vi "Dresden R2R Sputter 03.02.2018 IY24.vi"() -> ()   [LabVIEW 2009] (continued)
      tunnel: w5831 -> [w5835 w5844]
      tunnel: [w5835 w5842] -> w5828
      tunnel: w5830 -> [_ w5843]
      frame #0 {
      }
      frame #1 {
        n4043 = local read "Roll Status"() -> (w5841:T1)
        n4044 = Multiply(x=9.3, y=3.141592653589793) -> (x*y=w5838:dbl)
        n4045 = Multiply(x="RPM", y=6) -> (x*y=w5847:dbl)
        n4046 = Divide(x=w5843, y=u32 1000 ("milliseconds to wait")) -> (x/y=w5846:dbl)
        n4047 = Multiply(x=w5838, y="RPM") -> (x*y=→"Cevre":dbl)
        n4048 = Multiply(x=w5847, y=w5846) -> (x*y=w5845:dbl)
        n4049 = case shown="\"Backward\"" w5841 {
          tunnel: w5845 -> [w5856 w5863]
          tunnel: w5844 -> [w5855 w5862]
          tunnel: [w5852 w5857] -> w5842
          frame #0 {
            n4050 = Subtract(x=w5855, y=w5856) -> (x-y=w5851:dbl)
            n4051 = Less?(x=w5851, y=0.0) -> (x < y?=w5854:bool)
            n4052 = Select(t=360.0 ("y"), s=w5854, f=w5851) -> (s? t:f=w5852:dbl)
          }
          frame #1 {
            n4053 = Add(x=w5862, y=w5863) -> (x+y=w5858:dbl)
            n4054 = Less?(x=360.0 ("y"), y=w5858) -> (x < y?=w5861:bool)
            n4055 = Select(t=0.0 ("y"), s=w5861, f=w5858) -> (s? t:f=w5857:dbl)
          }
        }
      }
    }
    "Angle" <- w5828
    "Gauge" <- w5828
    n4056 = local read "Sim"() -> (w5829:bool)
  }
  n4057 = call <vilib>:"Read JPEG File.vi"("path to JPEG file"=w397) -> ("image data"=w396:T34)  [unwired: 8 in, 2 out]
  n4058 = call <vilib>:"Read JPEG File.vi"("path to JPEG file"=w398) -> ("image data"=w399:T34)  [unwired: 8 in, 2 out]
  n4059 = call <vilib>:"Read JPEG File.vi"("path to JPEG file"=w407) -> ("image data"=w406:T34)  [unwired: 8 in, 2 out]
  n4060 = call <vilib>:"Read JPEG File.vi"("path to JPEG file"=w313) -> ("image data"=w314:T34)  [unwired: 8 in, 2 out]
  n4061 = Build Path(base path="Gui_ch2_front_path", name or relative path="bv3 fail.jpg") -> (appended path=w114:path)
  n4062 = while {
    tunnel: w17 -> [w5874]
    tunnel: w16 -> [w5873]
    tunnel: [w5880] -> w15
    tunnel: [w5879] -> w14
    tunnel: data[3B] ("Serial Parameters") -> [w5868]
    stop <- FALSE stop-if-true
    # "Haberlesmenin sadece gerekli olan degerler ile\ndegilde tum degerler ile yapilmis olmasi\nhaberlesme hizini dusuruyor olabilir."
    n4063 = disable-structure shown="Enabled" {
      disable-tunnel: [w5912 w5934] -> w5877
      disable-tunnel: [w5911 w5936] -> w5876
      disable-tunnel: [w5910 w5938] -> w5875
      disable-tunnel: w5874 -> [w5909 w5947]
      disable-tunnel: w5873 -> [w5908 w5945]
      disable-tunnel: [w5907 w5944] -> w5872
      disable-tunnel: [w5906 w5946] -> w5871
      disable-tunnel: [w5905 w5948] -> w5870
      disable-tunnel: "Sim" -> [w5904 _]
      disable-tunnel: w5868 -> [w5903 w5948]
      disable-tunnel: [w5902 w5940] -> w5864
      frame #0 {
        n4064 = case shown="True" w5904 {
          tunnel: [w5928 "Sensor_DI Sim"] -> w5912
          tunnel: [w5927 "Sensor_DI Sim"] -> w5911
          tunnel: [w5926 "Sensor_DI Sim"] -> w5910
          tunnel: [w5925 "Sensor_DI Sim"] -> w5902
          tunnel: w5909 -> [w5924 w5932]
          tunnel: w5908 -> [w5923 w5931]
          tunnel: [w5922 w5931] -> w5907
          tunnel: [w5921 w5932] -> w5906
          tunnel: [w5913 w5929] -> w5905
          tunnel: w5903 -> [w5913 w5929]
          frame #0 {
            n4065 = call-poly <vilib>:"MB Serial Master Query (poly).vi"("VISA resource name"=w5924, "Starting Address"=u16 8, "Quantity"=u16 4, "error in"=w5923, "Serial Parameters"=w5913) -> ("VISA resource name out"=w5921:refnum<visa-resource-name>, "Discrete Inputs"=w5920:bool[], "error out"=w5922:errorcluster)  [unwired: 1 in, 11 out]
            n4066 = Index Array(array=w5920, index=0) -> (element=w5925:bool)
            n4067 = Index Array(array=w5920, index=1) -> (element=w5926:bool)
            n4068 = Index Array(array=w5920, index=2) -> (element=w5927:bool)
            n4069 = Index Array(array=w5920, index=3) -> (element=w5928:bool)
          }
          frame #1 {
          }
        }
      }
      frame #1 {
        n4070 = local read "Ch3_Motor_DO"() -> (→"Ch1_SRV_start_stop_do":bool)
        n4071 = call-poly <vilib>:"MB Serial Master Query (poly).vi"("VISA resource name"=w5947, "Starting Address"=u16 0, "Quantity"=u16 4, "error in"=w5945, "Serial Parameters"=w5948) -> ("VISA resource name out"=w5946:refnum<visa-resource-name>, "Discrete Inputs"=w5933:bool[], "error out"=w5944:errorcluster)  [unwired: 11 in, 1 out]
        n4072 = Index Array(array=w5933, index=3) -> (element=w5934:bool)
        n4073 = Index Array(array=w5933, index=2) -> (element=w5936:bool)
        n4074 = Index Array(array=w5933, index=1) -> (element=w5938:bool)
        n4075 = Index Array(array=w5933, index=0) -> (element=w5940:bool)
      }
    }
    "Ch1_Sensor_DI" <- w5864
    "Ch4_Sensor_DI" <- w5877
    "Ch2_Sensor_DI" <- w5875
    "Ch3_Sensor_DI" <- w5876
    "Ch1_SRV1_counter_di" <- w5864
    n4076 = Wait (ms)(milliseconds to wait=u32 5) -> ()  [unwired: 1 out]
    n4077 = local write "Sensor_DI Sim"(w5864) -> ()
    n4078 = disable-structure shown="Enabled" {
      disable-tunnel: "Ch1_Motor_DO" -> [w5893 w5900]
      disable-tunnel: [w5889 w5896] -> w5880
      disable-tunnel: [w5888 w5895] -> w5879
      disable-tunnel: w5872 -> [w5885 w5897]
      disable-tunnel: w5871 -> [w5884 w5898]
      disable-tunnel: w5870 -> [w5883 w5899]
      frame #0 {
        n4079 = Build Array(w5893, "Ch2_Motor_DO", "Ch3_Motor_DO", "Ch4_Motor_DO", "Motor_Dir_DO") -> (w5891:bool[])
        n4080 = call-poly <vilib>:"MB Serial Master Query (poly).vi"("VISA resource name"=w5884, "Starting Address"=u16 320, "Coils"=w5891, "error in"=w5885, "Serial Parameters"=w5883) -> ("VISA resource name out"=w5889:refnum<visa-resource-name>, "error out"=w5888:errorcluster)  [unwired: 12 in, 1 out]
      }
      frame #1 {
        n4081 = call-poly <vilib>:"MB Serial Master Query (poly).vi"("VISA resource name"=w5898, "Address"=u16 320 ("Starting Address"), "Coil"=w5900, "error in"=w5897, "Serial Parameters"=w5899) -> ("VISA resource name out"=w5896:refnum<visa-resource-name>, "error out"=w5895:errorcluster)  [unwired: 12 in, 1 out]
      }
    }
    n4082 = call "Elapsed Time145"() -> ("Elapsed Time (s)"=w5865:dbl)  [unwired: 12 in, 7 out]
    n4083 = feedback #121() -> (w5866:dbl)  [unwired: 1 in]
    n4084 = Subtract(x=w5865, y=w5866) -> (x-y=→"COM12 Loop Time":dbl)
  }
  n4085 = call <vilib>:"Read JPEG File.vi"("path to JPEG file"=w300) -> ("image data"=w299:T34)  [unwired: 8 in, 2 out]
  n4086 = call <vilib>:"Read JPEG File.vi"("path to JPEG file"=w410) -> ("image data"=w411:T34)  [unwired: 8 in, 2 out]
  n4087 = call <vilib>:"Read JPEG File.vi"("path to JPEG file"=w310) -> ("image data"=w309:T34)  [unwired: 8 in, 2 out]
  n4088 = Build Path(base path="Gui_ch2_front_path", name or relative path="bv3 on.jpg") -> (appended path=w117:path)
  n4089 = call <vilib>:"Read JPEG File.vi"("path to JPEG file"=w303) -> ("image data"=w304:T34)  [unwired: 8 in, 2 out]
  n4090 = Build Path(base path="Gui_ch2_top_path", name or relative path="atm3 fail.jpg") -> (appended path=w249:path)
  n4091 = Build Path(base path="Gui_ch2_front_path", name or relative path="gv front failled2.jpg") -> (appended path=w227:path)
  n4092 = call <vilib>:"Read JPEG File.vi"("path to JPEG file"=w106) -> ("image data"=w107:T34)  [unwired: 8 in, 2 out]
  n4093 = call <vilib>:"Read JPEG File.vi"("path to JPEG file"=w365) -> ("image data"=w364:T34)  [unwired: 8 in, 2 out]
  n4094 = call <vilib>:"Read JPEG File.vi"("path to JPEG file"=w149) -> ("image data"=w150:T34)  [unwired: 8 in, 2 out]
  n4095 = Build Path(base path="Gui_ch2_top_path", name or relative path="atm3 on.jpg") -> (appended path=w250:path)
  n4096 = Build Path(base path="Gui_ch2_top_path", name or relative path="pg2 fail.jpg") -> (appended path=w254:path)
  n4097 = Build Path(base path="Gui_ch2_top_path", name or relative path="cc fail.jpg") -> (appended path=w261:path)
  n4098 = Build Path(base path="Gui_ch2_top_path", name or relative path="pg2 fail.jpg") -> (appended path=w267:path)
  n4099 = call <vilib>:"Read JPEG File.vi"("path to JPEG file"=w473) -> ("image data"=w472:T34)  [unwired: 8 in, 2 out]
  n4100 = call <vilib>:"Read JPEG File.vi"("path to JPEG file"=w477) -> ("image data"=w478:T34)  [unwired: 8 in, 2 out]
  n4101 = Build Path(base path="Gui_ch2_top_path", name or relative path="pg2 on.jpg") -> (appended path=w253:path)
  n4102 = Build Path(base path="Gui_ch2_top_path", name or relative path="cc on.jpg") -> (appended path=w262:path)
  n4103 = Build Path(base path="Gui_ch2_top_path", name or relative path="pg2 on.jpg") -> (appended path=w268:path)
  n4104 = call <vilib>:"Read JPEG File.vi"("path to JPEG file"=w103) -> ("image data"=w102:T34)  [unwired: 8 in, 2 out]
  n4105 = call <vilib>:"Read JPEG File.vi"("path to JPEG file"=w537) -> ("image data"=w536:T34)  [unwired: 8 in, 2 out]
  n4106 = call <vilib>:"Read JPEG File.vi"("path to JPEG file"=w368) -> ("image data"=w369:T34)  [unwired: 8 in, 2 out]
  n4107 = call <vilib>:"Read JPEG File.vi"("path to JPEG file"=w487) -> ("image data"=w488:T34)  [unwired: 8 in, 2 out]
  n4108 = call <vilib>:"Read JPEG File.vi"("path to JPEG file"=w474) -> ("image data"=w475:T34)  [unwired: 8 in, 2 out]
  n4109 = call <vilib>:"Read JPEG File.vi"("path to JPEG file"=w146) -> ("image data"=w145:T34)  [unwired: 8 in, 2 out]
  n4110 = Build Path(base path="Gui_ch2_top_path", name or relative path="bv1 fail.jpg") -> (appended path=w272:path)
  n4111 = Build Path(base path="Gui_ch2_front_path", name or relative path="gv front open2.jpg") -> (appended path=w230:path)
  n4112 = call <vilib>:"Read JPEG File.vi"("path to JPEG file"=w538) -> ("image data"=w539:T34)  [unwired: 8 in, 2 out]
  n4113 = call <vilib>:"Read JPEG File.vi"("path to JPEG file"=w527) -> ("image data"=w526:T34)  [unwired: 8 in, 2 out]
  n4114 = call <vilib>:"Read JPEG File.vi"("path to JPEG file"=w499) -> ("image data"=w498:T34)  [unwired: 8 in, 2 out]
  n4115 = Build Path(base path="Gui_ch2_top_path", name or relative path="chamber 2 top piston open.jpg") -> (appended path=w485:path)
  n4116 = Build Path(base path="Gui_ch2_top_path", name or relative path="bv1 on.jpg") -> (appended path=w271:path)
  n4117 = Build Path(base path="Gui_ch2_top_path", name or relative path="atm3 fail.jpg") -> (appended path=w220:path)
  n4118 = call <vilib>:"Read JPEG File.vi"("path to JPEG file"=w500) -> ("image data"=w501:T34)  [unwired: 8 in, 2 out]
  n4119 = call <vilib>:"Read JPEG File.vi"("path to JPEG file"=w480) -> ("image data"=w479:T34)  [unwired: 8 in, 2 out]
  n4120 = Build Path(base path="Gui_ch2_top_path", name or relative path="chamber 2 top piston failed.jpg") -> (appended path=w492:path)
  n4121 = Build Path(base path="Gui_ch2_top_path", name or relative path="atm3 on.jpg") -> (appended path=w219:path)
  n4122 = Build Path(base path="Gui_ch2_top_path", name or relative path="pg2 fail.jpg") -> (appended path=w215:path)
  n4123 = Build Path(base path="Gui_ch2_top_path", name or relative path="cc fail.jpg") -> (appended path=w208:path)
  n4124 = Build Path(base path="Gui_ch2_top_path", name or relative path="pg2 fail.jpg") -> (appended path=w202:path)
  n4125 = Build Path(base path="Gui_ch2_top_path", name or relative path="gv top failed2.jpg") -> (appended path=w288:path)
  n4126 = Build Path(base path="Gui_ch2_top_path", name or relative path="pg2 on.jpg") -> (appended path=w216:path)
  n4127 = Build Path(base path="Gui_ch2_top_path", name or relative path="cc on.jpg") -> (appended path=w207:path)
  n4128 = Build Path(base path="Gui_ch2_top_path", name or relative path="pg2 on.jpg") -> (appended path=w201:path)
  n4129 = call <vilib>:"Read JPEG File.vi"("path to JPEG file"=w483) -> ("image data"=w484:T34)  [unwired: 8 in, 2 out]
  n4130 = Build Path(base path="Gui_ch2_top_path", name or relative path="chamber 2 top piston open.jpg") -> (appended path=w429:path)
  n4131 = Build Path(base path="Gui_ch2_top_path", name or relative path="bv1 fail.jpg") -> (appended path=w197:path)
  n4132 = Build Path(base path="Gui_ch2_top_path", name or relative path="gv top open.jpg") -> (appended path=w466:path)
  n4133 = Build Path(base path="Gui_ch2_top_path", name or relative path="gv top open2.jpg") -> (appended path=w294:path)
  n4134 = Build Path(base path="Gui_ch2_top_path", name or relative path="chamber 2 top piston failed.jpg") -> (appended path=w427:path)
  n4135 = Build Path(base path="Gui_ch2_top_path", name or relative path="bv1 on.jpg") -> (appended path=w198:path)
  n4136 = Build Path(base path="Gui_ch2_top_path", name or relative path="gv top failed.jpg") -> (appended path=w465:path)
  n4137 = Build Path(base path="Gui_ch2_top_path", name or relative path="gv front failled2.jpg") -> (appended path=w181:path)
  n4138 = call <vilib>:"Read JPEG File.vi"("path to JPEG file"=w390) -> ("image data"=w391:T34)  [unwired: 8 in, 2 out]
  n4139 = Build Path(base path="Gui_ch1_top_path", name or relative path="chamber 4 top piston open.jpg") -> (appended path=w415:path)
  n4140 = Build Path(base path="Gui_ch2_top_path", name or relative path="gv top open.jpg") -> (appended path=w433:path)
  n4141 = call <vilib>:"Read JPEG File.vi"("path to JPEG file"=w389) -> ("image data"=w388:T34)  [unwired: 8 in, 2 out]
  n4142 = call <vilib>:"Read JPEG File.vi"("path to JPEG file"=w400) -> ("image data"=w401:T34)  [unwired: 8 in, 2 out]
  n4143 = Build Path(base path="Gui_ch1_top_path", name or relative path="chamber 4 top piston failed.jpg") -> (appended path=w416:path)
  n4144 = Build Path(base path="Gui_ch2_top_path", name or relative path="gv top failed.jpg") -> (appended path=w434:path)
  n4145 = Build Path(base path="Gui_ch2_top_path", name or relative path="gv front open2.jpg") -> (appended path=w177:path)
  n4146 = call <vilib>:"Unflatten Pixmap.vi"("image data"=w463) -> ("24-bit pixmap"=w557:u32[][])  [unwired: 4 in, 6 out]
  n4147 = Build Path(base path="Gui_ch1_top_path", name or relative path="bv3 fail.jpg") -> (appended path=w94:path)
  n4148 = call <vilib>:"Read JPEG File.vi"("path to JPEG file"=w359) -> ("image data"=w360:T34)  [unwired: 8 in, 2 out]
  n4149 = Build Path(base path="Gui_ch1_top_path", name or relative path="gv top open2.jpg") -> (appended path=w420:path)
  n4150 = Build Path(base path="Gui_ch1_top_path", name or relative path="bv3 on.jpg") -> (appended path=w97:path)
  n4151 = Build Path(base path="Gui_ch1_top_path", name or relative path="gv top failed2.jpg") -> (appended path=w419:path)
  n4152 = call <vilib>:"Read JPEG File.vi"("path to JPEG file"=w356) -> ("image data"=w355:T34)  [unwired: 8 in, 2 out]
  n4153 = call <vilib>:"Read JPEG File.vi"("path to JPEG file"=w276) -> ("image data"=w275:T34)  [unwired: 8 in, 2 out]
  n4154 = Build Path(base path="Gui_ch1_top_path", name or relative path="atm3 fail.jpg") -> (appended path=w64:path)
  n4155 = call <vilib>:"Read JPEG File.vi"("path to JPEG file"=w512) -> ("image data"=w513:T34)  [unwired: 8 in, 2 out]
  n4156 = call <vilib>:"Read JPEG File.vi"("path to JPEG file"=w286) -> ("image data"=w287:T34)  [unwired: 8 in, 2 out]
  n4157 = call <vilib>:"Read JPEG File.vi"("path to JPEG file"=w511) -> ("image data"=w510:T34)  [unwired: 8 in, 2 out]
  n4158 = call <vilib>:"Read JPEG File.vi"("path to JPEG file"=w279) -> ("image data"=w280:T34)  [unwired: 8 in, 2 out]
  n4159 = call <vilib>:"Read JPEG File.vi"("path to JPEG file"=w349) -> ("image data"=w350:T34)  [unwired: 8 in, 2 out]
  n4160 = call <vilib>:"Read JPEG File.vi"("path to JPEG file"=w283) -> ("image data"=w282:T34)  [unwired: 8 in, 2 out]
  n4161 = call <vilib>:"Read JPEG File.vi"("path to JPEG file"=w456) -> ("image data"=w457:T34)  [unwired: 8 in, 2 out]
  n4162 = call <vilib>:"Read JPEG File.vi"("path to JPEG file"=w452) -> ("image data"=w451:T34)  [unwired: 8 in, 2 out]
  n4163 = Build Path(base path="Gui_ch1_top_path", name or relative path="atm3 on.jpg") -> (appended path=w65:path)
  n4164 = Build Path(base path="Gui_ch1_top_path", name or relative path="pg2 fail.jpg") -> (appended path=w69:path)
  n4165 = Build Path(base path="Gui_ch1_top_path", name or relative path="cc fail.jpg") -> (appended path=w76:path)
  n4166 = Build Path(base path="Gui_ch1_top_path", name or relative path="pg2 fail.jpg") -> (appended path=w82:path)
  n4167 = Build Path(base path="Gui_ch1_top_path", name or relative path="sov on.jpg") -> (appended path=w39:path)
  n4168 = call <vilib>:"Read JPEG File.vi"("path to JPEG file"=w348) -> ("image data"=w347:T34)  [unwired: 8 in, 2 out]
  n4169 = call <vilib>:"Read JPEG File.vi"("path to JPEG file"=w340) -> ("image data"=w339:T34)  [unwired: 8 in, 2 out]
  n4170 = call <vilib>:"Read JPEG File.vi"("path to JPEG file"=w333) -> ("image data"=w334:T34)  [unwired: 8 in, 2 out]
  n4171 = call <vilib>:"Read JPEG File.vi"("path to JPEG file"=w325) -> ("image data"=w326:T34)  [unwired: 8 in, 2 out]
  n4172 = call <vilib>:"Read JPEG File.vi"("path to JPEG file"=w155) -> ("image data"=w154:T34)  [unwired: 8 in, 2 out]
  n4173 = call <vilib>:"Read JPEG File.vi"("path to JPEG file"=w444) -> ("image data"=w443:T34)  [unwired: 8 in, 2 out]
  n4174 = call <vilib>:"Read JPEG File.vi"("path to JPEG file"=w455) -> ("image data"=w454:T34)  [unwired: 8 in, 2 out]
  n4175 = Build Path(base path="Gui_ch2_front_path", name or relative path="bv2 on.jpg") -> (appended path=w120:path)
  n4176 = call <vilib>:"Read JPEG File.vi"("path to JPEG file"=w193) -> ("image data"=w194:T34)  [unwired: 8 in, 2 out]
  n4177 = Build Path(base path="Gui_ch1_top_path", name or relative path="pg2 on.jpg") -> (appended path=w68:path)
  n4178 = Build Path(base path="Gui_ch1_top_path", name or relative path="cc on.jpg") -> (appended path=w77:path)
  n4179 = Build Path(base path="Gui_ch1_top_path", name or relative path="pg2 on.jpg") -> (appended path=w83:path)
  n4180 = Build Path(base path="Gui_ch1_top_path", name or relative path="sov fail.jpg") -> (appended path=w40:path)
  n4181 = call <vilib>:"Read JPEG File.vi"("path to JPEG file"=w341) -> ("image data"=w342:T34)  [unwired: 8 in, 2 out]
  n4182 = call <vilib>:"Read JPEG File.vi"("path to JPEG file"=w332) -> ("image data"=w331:T34)  [unwired: 8 in, 2 out]
  n4183 = call <vilib>:"Read JPEG File.vi"("path to JPEG file"=w324) -> ("image data"=w323:T34)  [unwired: 8 in, 2 out]
  n4184 = call <vilib>:"Read JPEG File.vi"("path to JPEG file"=w438) -> ("image data"=w439:T34)  [unwired: 8 in, 2 out]
  n4185 = Build Path(base path="Gui_ch2_front_path", name or relative path="bv2 fail.jpg") -> (appended path=w121:path)
  n4186 = call <vilib>:"Read JPEG File.vi"("path to JPEG file"="Background_ch2_top_path") -> ("image data"=w460:T34)  [unwired: 8 in, 2 out]
  n4187 = call <vilib>:"Read JPEG File.vi"("path to JPEG file"=w183) -> ("image data"=w182:T34)  [unwired: 8 in, 2 out]
  n4188 = Build Path(base path="Gui_ch1_top_path", name or relative path="bv1 fail.jpg") -> (appended path=w87:path)
  n4189 = call <vilib>:"Read JPEG File.vi"("path to JPEG file"=w318) -> ("image data"=w305:T34)  [unwired: 8 in, 2 out]
  n4190 = call <vilib>:"Read JPEG File.vi"("path to JPEG file"=w158) -> ("image data"=w159:T34)  [unwired: 8 in, 2 out]
  n4191 = call <vilib>:"Read JPEG File.vi"("path to JPEG file"=w437) -> ("image data"=w436:T34)  [unwired: 8 in, 2 out]
  n4192 = call <vilib>:"Read JPEG File.vi"("path to JPEG file"=w449) -> ("image data"=w450:T34)  [unwired: 8 in, 2 out]
  n4193 = call <vilib>:"Read JPEG File.vi"("path to JPEG file"=w190) -> ("image data"=w189:T34)  [unwired: 8 in, 2 out]
  n4194 = Build Path(base path="Gui_ch1_top_path", name or relative path="bv1 on.jpg") -> (appended path=w86:path)
  n4195 = call <vilib>:"Read JPEG File.vi"("path to JPEG file"=w507) -> ("image data"=w506:T34)  [unwired: 8 in, 2 out]
  n4196 = call <vilib>:"Read JPEG File.vi"("path to JPEG file"=w319) -> ("image data"=w320:T34)  [unwired: 8 in, 2 out]
  n4197 = call <vilib>:"Read JPEG File.vi"("path to JPEG file"=w186) -> ("image data"=w187:T34)  [unwired: 8 in, 2 out]
  n4198 = call <vilib>:"Unflatten Pixmap.vi"("image data"=w522) -> ("24-bit pixmap"=w578:u32[][])  [unwired: 4 in, 6 out]
  n4199 = call <vilib>:"Read JPEG File.vi"("path to JPEG file"=w508) -> ("image data"=w509:T34)  [unwired: 8 in, 2 out]
  n4200 = call <vilib>:"Read JPEG File.vi"("path to JPEG file"=w446) -> ("image data"=w445:T34)  [unwired: 8 in, 2 out]
  n4201 = call <vilib>:"Read JPEG File.vi"("path to JPEG file"=w141) -> ("image data"=w142:T34)  [unwired: 8 in, 2 out]
  n4202 = call <vilib>:"Unflatten Pixmap.vi"("image data"=w531) -> ("24-bit pixmap"=w581:u32[][])  [unwired: 4 in, 6 out]
  n4203 = call <vilib>:"Read JPEG File.vi"("path to JPEG file"=w140) -> ("image data"=w139:T34)  [unwired: 8 in, 2 out]
  n4204 = call <vilib>:"Unflatten Pixmap.vi"("image data"=w528) -> ("24-bit pixmap"=w579:u32[][])  [unwired: 4 in, 6 out]
  n4205 = call <vilib>:"Unflatten Pixmap.vi"("image data"=w521) -> ("24-bit pixmap"=w577:u32[][])  [unwired: 4 in, 6 out]
  n4206 = call <vilib>:"Read JPEG File.vi"("path to JPEG file"=w129) -> ("image data"=w128:T34)  [unwired: 8 in, 2 out]
  n4207 = call <vilib>:"Unflatten Pixmap.vi"("image data"=w516) -> ("24-bit pixmap"=w576:u32[][])  [unwired: 4 in, 6 out]
  n4208 = call <vilib>:"Read JPEG File.vi"("path to JPEG file"=w132) -> ("image data"=w133:T34)  [unwired: 8 in, 2 out]
  n4209 = call <vilib>:"Unflatten Pixmap.vi"("image data"=w405) -> ("24-bit pixmap"=w377:u32[][])  [unwired: 4 in, 6 out]
  n4210 = call <vilib>:"Unflatten Pixmap.vi"("image data"=w396) -> ("24-bit pixmap"=w374:u32[][])  [unwired: 4 in, 6 out]
  n4211 = call <vilib>:"Unflatten Pixmap.vi"("image data"=w399) -> ("24-bit pixmap"=w376:u32[][])  [unwired: 4 in, 6 out]
  n4212 = call <vilib>:"Unflatten Pixmap.vi"("image data"=w406) -> ("24-bit pixmap"=w378:u32[][])  [unwired: 4 in, 6 out]
  n4213 = call <vilib>:"Unflatten Pixmap.vi"("image data"=w314) -> ("24-bit pixmap"=w308:u32[][])  [unwired: 4 in, 6 out]
  n4214 = call <vilib>:"Unflatten Pixmap.vi"("image data"=w299) -> ("24-bit pixmap"=w296:u32[][])  [unwired: 4 in, 6 out]
  n4215 = call <vilib>:"Unflatten Pixmap.vi"("image data"=w411) -> ("24-bit pixmap"=w379:u32[][])  [unwired: 4 in, 6 out]
  n4216 = call <vilib>:"Unflatten Pixmap.vi"("image data"=w309) -> ("24-bit pixmap"=w307:u32[][])  [unwired: 4 in, 6 out]
  n4217 = call <vilib>:"Unflatten Pixmap.vi"("image data"=w304) -> ("24-bit pixmap"=w297:u32[][])  [unwired: 4 in, 6 out]
  n4218 = call <vilib>:"Unflatten Pixmap.vi"("image data"=w107) -> ("24-bit pixmap"=w101:u32[][])  [unwired: 4 in, 6 out]
  n4219 = call <vilib>:"Unflatten Pixmap.vi"("image data"=w364) -> ("24-bit pixmap"=w362:u32[][])  [unwired: 4 in, 6 out]
  n4220 = call <vilib>:"Unflatten Pixmap.vi"("image data"=w150) -> ("24-bit pixmap"=w144:u32[][])  [unwired: 4 in, 6 out]
  n4221 = call <vilib>:"Unflatten Pixmap.vi"("image data"=w472) -> ("24-bit pixmap"=w564:u32[][])  [unwired: 4 in, 6 out]
  n4222 = call <vilib>:"Unflatten Pixmap.vi"("image data"=w478) -> ("24-bit pixmap"=w562:u32[][])  [unwired: 4 in, 6 out]
  n4223 = call <vilib>:"Unflatten Pixmap.vi"("image data"=w102) -> ("24-bit pixmap"=w100:u32[][])  [unwired: 4 in, 6 out]
  n4224 = call <vilib>:"Unflatten Pixmap.vi"("image data"=w536) -> ("24-bit pixmap"=w583:u32[][])  [unwired: 4 in, 6 out]
  n4225 = call <vilib>:"Unflatten Pixmap.vi"("image data"=w369) -> ("24-bit pixmap"=w363:u32[][])  [unwired: 4 in, 6 out]
  n4226 = call <vilib>:"Unflatten Pixmap.vi"("image data"=w488) -> ("24-bit pixmap"=w565:u32[][])  [unwired: 4 in, 6 out]
  n4227 = call <vilib>:"Unflatten Pixmap.vi"("image data"=w475) -> ("24-bit pixmap"=w563:u32[][])  [unwired: 4 in, 6 out]
  n4228 = call <vilib>:"Unflatten Pixmap.vi"("image data"=w145) -> ("24-bit pixmap"=w143:u32[][])  [unwired: 4 in, 6 out]
  n4229 = call <vilib>:"Read JPEG File.vi"("path to JPEG file"=w114) -> ("image data"=w113:T34)  [unwired: 8 in, 2 out]
  n4230 = call <vilib>:"Unflatten Pixmap.vi"("image data"=w539) -> ("24-bit pixmap"=w582:u32[][])  [unwired: 4 in, 6 out]
  n4231 = call <vilib>:"Unflatten Pixmap.vi"("image data"=w526) -> ("24-bit pixmap"=w580:u32[][])  [unwired: 4 in, 6 out]
  n4232 = call <vilib>:"Unflatten Pixmap.vi"("image data"=w498) -> ("24-bit pixmap"=w570:u32[][])  [unwired: 4 in, 6 out]
  n4233 = call <vilib>:"Unflatten Pixmap.vi"("image data"=w501) -> ("24-bit pixmap"=w569:u32[][])  [unwired: 4 in, 6 out]
  n4234 = call <vilib>:"Unflatten Pixmap.vi"("image data"=w479) -> ("24-bit pixmap"=w561:u32[][])  [unwired: 4 in, 6 out]
  n4235 = call <vilib>:"Read JPEG File.vi"("path to JPEG file"=w117) -> ("image data"=w118:T34)  [unwired: 8 in, 2 out]
  n4236 = call <vilib>:"Unflatten Pixmap.vi"("image data"=w484) -> ("24-bit pixmap"=w560:u32[][])  [unwired: 4 in, 6 out]
  n4237 = call <vilib>:"Read JPEG File.vi"("path to JPEG file"=w249) -> ("image data"=w248:T34)  [unwired: 8 in, 2 out]
  n4238 = call <vilib>:"Read JPEG File.vi"("path to JPEG file"=w227) -> ("image data"=w226:T34)  [unwired: 8 in, 2 out]
  n4239 = call <vilib>:"Read JPEG File.vi"("path to JPEG file"=w250) -> ("image data"=w251:T34)  [unwired: 8 in, 2 out]
  n4240 = call <vilib>:"Read JPEG File.vi"("path to JPEG file"=w254) -> ("image data"=w255:T34)  [unwired: 8 in, 2 out]
  n4241 = call <vilib>:"Read JPEG File.vi"("path to JPEG file"=w261) -> ("image data"=w260:T34)  [unwired: 8 in, 2 out]
  n4242 = call <vilib>:"Read JPEG File.vi"("path to JPEG file"=w267) -> ("image data"=w266:T34)  [unwired: 8 in, 2 out]
  n4243 = call <vilib>:"Read JPEG File.vi"("path to JPEG file"=w485) -> ("image data"=w486:T34)  [unwired: 8 in, 2 out]
  n4244 = call <vilib>:"Read JPEG File.vi"("path to JPEG file"=w253) -> ("image data"=w252:T34)  [unwired: 8 in, 2 out]
  n4245 = call <vilib>:"Read JPEG File.vi"("path to JPEG file"=w262) -> ("image data"=w263:T34)  [unwired: 8 in, 2 out]
  n4246 = call <vilib>:"Read JPEG File.vi"("path to JPEG file"=w268) -> ("image data"=w269:T34)  [unwired: 8 in, 2 out]
  n4247 = call <vilib>:"Read JPEG File.vi"("path to JPEG file"=w288) -> ("image data"=w289:T34)  [unwired: 8 in, 2 out]
  n4248 = call <vilib>:"Read JPEG File.vi"("path to JPEG file"=w272) -> ("image data"=w281:T34)  [unwired: 8 in, 2 out]
  n4249 = call <vilib>:"Read JPEG File.vi"("path to JPEG file"=w230) -> ("image data"=w231:T34)  [unwired: 8 in, 2 out]
  n4250 = call <vilib>:"Unflatten Pixmap.vi"("image data"=w391) -> ("24-bit pixmap"=w372:u32[][])  [unwired: 4 in, 6 out]
  n4251 = call <vilib>:"Read JPEG File.vi"("path to JPEG file"=w271) -> ("image data"=w270:T34)  [unwired: 8 in, 2 out]
  n4252 = call <vilib>:"Read JPEG File.vi"("path to JPEG file"=w220) -> ("image data"=w221:T34)  [unwired: 8 in, 2 out]
  n4253 = call <vilib>:"Unflatten Pixmap.vi"("image data"=w388) -> ("24-bit pixmap"=w373:u32[][])  [unwired: 4 in, 6 out]
  n4254 = call <vilib>:"Unflatten Pixmap.vi"("image data"=w401) -> ("24-bit pixmap"=w375:u32[][])  [unwired: 4 in, 6 out]
  n4255 = call <vilib>:"Read JPEG File.vi"("path to JPEG file"=w492) -> ("image data"=w493:T34)  [unwired: 8 in, 2 out]
  n4256 = call <vilib>:"Read JPEG File.vi"("path to JPEG file"=w429) -> ("image data"=w428:T34)  [unwired: 8 in, 2 out]
  n4257 = call <vilib>:"Read JPEG File.vi"("path to JPEG file"=w219) -> ("image data"=w218:T34)  [unwired: 8 in, 2 out]
  n4258 = call <vilib>:"Read JPEG File.vi"("path to JPEG file"=w215) -> ("image data"=w214:T34)  [unwired: 8 in, 2 out]
  n4259 = call <vilib>:"Read JPEG File.vi"("path to JPEG file"=w208) -> ("image data"=w209:T34)  [unwired: 8 in, 2 out]
  n4260 = call <vilib>:"Read JPEG File.vi"("path to JPEG file"=w202) -> ("image data"=w203:T34)  [unwired: 8 in, 2 out]
  n4261 = call <vilib>:"Read JPEG File.vi"("path to JPEG file"=w216) -> ("image data"=w217:T34)  [unwired: 8 in, 2 out]
  n4262 = call <vilib>:"Read JPEG File.vi"("path to JPEG file"=w207) -> ("image data"=w206:T34)  [unwired: 8 in, 2 out]
  n4263 = call <vilib>:"Read JPEG File.vi"("path to JPEG file"=w201) -> ("image data"=w200:T34)  [unwired: 8 in, 2 out]
  n4264 = call <vilib>:"Read JPEG File.vi"("path to JPEG file"=w181) -> ("image data"=w180:T34)  [unwired: 8 in, 2 out]
  n4265 = call <vilib>:"Read JPEG File.vi"("path to JPEG file"=w197) -> ("image data"=w188:T34)  [unwired: 8 in, 2 out]
  n4266 = call <vilib>:"Read JPEG File.vi"("path to JPEG file"=w466) -> ("image data"=w467:T34)  [unwired: 8 in, 2 out]
  n4267 = call <vilib>:"Read JPEG File.vi"("path to JPEG file"=w294) -> ("image data"=w295:T34)  [unwired: 8 in, 2 out]
  n4268 = call <vilib>:"Read JPEG File.vi"("path to JPEG file"=w427) -> ("image data"=w426:T34)  [unwired: 8 in, 2 out]
  n4269 = call <vilib>:"Read JPEG File.vi"("path to JPEG file"=w198) -> ("image data"=w199:T34)  [unwired: 8 in, 2 out]
  n4270 = call <vilib>:"Unflatten Pixmap.vi"("image data"=w360) -> ("24-bit pixmap"=w354:u32[][])  [unwired: 4 in, 6 out]
  n4271 = call <vilib>:"Read JPEG File.vi"("path to JPEG file"=w465) -> ("image data"=w464:T34)  [unwired: 8 in, 2 out]
  n4272 = call <vilib>:"Read JPEG File.vi"("path to JPEG file"=w415) -> ("image data"=w414:T34)  [unwired: 8 in, 2 out]
  n4273 = call <vilib>:"Unflatten Pixmap.vi"("image data"=w355) -> ("24-bit pixmap"=w353:u32[][])  [unwired: 4 in, 6 out]
  n4274 = call <vilib>:"Read JPEG File.vi"("path to JPEG file"=w433) -> ("image data"=w432:T34)  [unwired: 8 in, 2 out]
  n4275 = call <vilib>:"Read JPEG File.vi"("path to JPEG file"=w416) -> ("image data"=w417:T34)  [unwired: 8 in, 2 out]
  n4276 = call <vilib>:"Read JPEG File.vi"("path to JPEG file"=w434) -> ("image data"=w435:T34)  [unwired: 8 in, 2 out]
  n4277 = call <vilib>:"Read JPEG File.vi"("path to JPEG file"=w177) -> ("image data"=w176:T34)  [unwired: 8 in, 2 out]
  n4278 = call <vilib>:"Read JPEG File.vi"("path to JPEG file"=w94) -> ("image data"=w93:T34)  [unwired: 8 in, 2 out]
  n4279 = call <vilib>:"Unflatten Pixmap.vi"("image data"=w275) -> ("24-bit pixmap"=w239:u32[][])  [unwired: 4 in, 6 out]
  n4280 = call <vilib>:"Read JPEG File.vi"("path to JPEG file"=w420) -> ("image data"=w421:T34)  [unwired: 8 in, 2 out]
  n4281 = call <vilib>:"Read JPEG File.vi"("path to JPEG file"=w97) -> ("image data"=w98:T34)  [unwired: 8 in, 2 out]
  n4282 = call <vilib>:"Unflatten Pixmap.vi"("image data"=w513) -> ("24-bit pixmap"=w574:u32[][])  [unwired: 4 in, 6 out]
  n4283 = call <vilib>:"Unflatten Pixmap.vi"("image data"=w287) -> ("24-bit pixmap"=w237:u32[][])  [unwired: 4 in, 6 out]
  n4284 = call <vilib>:"Read JPEG File.vi"("path to JPEG file"=w419) -> ("image data"=w418:T34)  [unwired: 8 in, 2 out]
  n4285 = call <vilib>:"Unflatten Pixmap.vi"("image data"=w510) -> ("24-bit pixmap"=w575:u32[][])  [unwired: 4 in, 6 out]
  n4286 = call <vilib>:"Unflatten Pixmap.vi"("image data"=w280) -> ("24-bit pixmap"=w238:u32[][])  [unwired: 4 in, 6 out]
  n4287 = call <vilib>:"Unflatten Pixmap.vi"("image data"=w350) -> ("24-bit pixmap"=w346:u32[][])  [unwired: 4 in, 6 out]
  n4288 = call <vilib>:"Unflatten Pixmap.vi"("image data"=w282) -> ("24-bit pixmap"=w236:u32[][])  [unwired: 4 in, 6 out]
  n4289 = call <vilib>:"Unflatten Pixmap.vi"("image data"=w457) -> ("24-bit pixmap"=w553:u32[][])  [unwired: 4 in, 6 out]
  n4290 = call <vilib>:"Unflatten Pixmap.vi"("image data"=w451) -> ("24-bit pixmap"=w551:u32[][])  [unwired: 4 in, 6 out]
  n4291 = call <vilib>:"Unflatten Pixmap.vi"("image data"=w347) -> ("24-bit pixmap"=w345:u32[][])  [unwired: 4 in, 6 out]
  n4292 = call <vilib>:"Unflatten Pixmap.vi"("image data"=w339) -> ("24-bit pixmap"=w343:u32[][])  [unwired: 4 in, 6 out]
  n4293 = call <vilib>:"Unflatten Pixmap.vi"("image data"=w334) -> ("24-bit pixmap"=w330:u32[][])  [unwired: 4 in, 6 out]
  n4294 = call <vilib>:"Unflatten Pixmap.vi"("image data"=w326) -> ("24-bit pixmap"=w322:u32[][])  [unwired: 4 in, 6 out]
  n4295 = call <vilib>:"Unflatten Pixmap.vi"("image data"=w154) -> ("24-bit pixmap"=w152:u32[][])  [unwired: 4 in, 6 out]
  n4296 = call <vilib>:"Unflatten Pixmap.vi"("image data"=w443) -> ("24-bit pixmap"=w554:u32[][])  [unwired: 4 in, 6 out]
  n4297 = call <vilib>:"Unflatten Pixmap.vi"("image data"=w454) -> ("24-bit pixmap"=w552:u32[][])  [unwired: 4 in, 6 out]
  n4298 = call <vilib>:"Unflatten Pixmap.vi"("image data"=w194) -> ("24-bit pixmap"=w163:u32[][])  [unwired: 4 in, 6 out]
  n4299 = call <vilib>:"Unflatten Pixmap.vi"("image data"=w342) -> ("24-bit pixmap"=w344:u32[][])  [unwired: 4 in, 6 out]
  n4300 = call <vilib>:"Unflatten Pixmap.vi"("image data"=w331) -> ("24-bit pixmap"=w329:u32[][])  [unwired: 4 in, 6 out]
  n4301 = call <vilib>:"Unflatten Pixmap.vi"("image data"=w323) -> ("24-bit pixmap"=w321:u32[][])  [unwired: 4 in, 6 out]
  n4302 = call <vilib>:"Unflatten Pixmap.vi"("image data"=w439) -> ("24-bit pixmap"=w556:u32[][])  [unwired: 4 in, 6 out]
  n4303 = call <vilib>:"Unflatten Pixmap.vi"("image data"=w460) -> ("24-bit pixmap"=w548:u32[][])  [unwired: 4 in, 6 out]
  n4304 = call <vilib>:"Unflatten Pixmap.vi"("image data"=w182) -> ("24-bit pixmap"=w161:u32[][])  [unwired: 4 in, 6 out]
  n4305 = call <vilib>:"Unflatten Pixmap.vi"("image data"=w159) -> ("24-bit pixmap"=w151:u32[][])  [unwired: 4 in, 6 out]
  n4306 = call <vilib>:"Unflatten Pixmap.vi"("image data"=w436) -> ("24-bit pixmap"=w555:u32[][])  [unwired: 4 in, 6 out]
  n4307 = call <vilib>:"Unflatten Pixmap.vi"("image data"=w450) -> ("24-bit pixmap"=w550:u32[][])  [unwired: 4 in, 6 out]
  n4308 = call <vilib>:"Unflatten Pixmap.vi"("image data"=w189) -> ("24-bit pixmap"=w162:u32[][])  [unwired: 4 in, 6 out]
  n4309 = call <vilib>:"Unflatten Pixmap.vi"("image data"=w506) -> ("24-bit pixmap"=w572:u32[][])  [unwired: 4 in, 6 out]
  n4310 = call <vilib>:"Unflatten Pixmap.vi"("image data"=w320) -> ("24-bit pixmap"=w315:u32[][])  [unwired: 4 in, 6 out]
  n4311 = call <vilib>:"Unflatten Pixmap.vi"("image data"=w187) -> ("24-bit pixmap"=w160:u32[][])  [unwired: 4 in, 6 out]
  n4312 = call <vilib>:"Read JPEG File.vi"("path to JPEG file"=w64) -> ("image data"=w63:T34)  [unwired: 8 in, 2 out]
  n4313 = call <vilib>:"Unflatten Pixmap.vi"("image data"=w509) -> ("24-bit pixmap"=w573:u32[][])  [unwired: 4 in, 6 out]
  n4314 = call <vilib>:"Unflatten Pixmap.vi"("image data"=w445) -> ("24-bit pixmap"=w549:u32[][])  [unwired: 4 in, 6 out]
  n4315 = call <vilib>:"Unflatten Pixmap.vi"("image data"=w142) -> ("24-bit pixmap"=w138:u32[][])  [unwired: 4 in, 6 out]
  n4316 = call <vilib>:"Unflatten Pixmap.vi"("image data"=w139) -> ("24-bit pixmap"=w137:u32[][])  [unwired: 4 in, 6 out]
  n4317 = call <vilib>:"Read JPEG File.vi"("path to JPEG file"=w65) -> ("image data"=w66:T34)  [unwired: 8 in, 2 out]
  n4318 = call <vilib>:"Read JPEG File.vi"("path to JPEG file"=w69) -> ("image data"=w70:T34)  [unwired: 8 in, 2 out]
  n4319 = call <vilib>:"Read JPEG File.vi"("path to JPEG file"=w76) -> ("image data"=w75:T34)  [unwired: 8 in, 2 out]
  n4320 = call <vilib>:"Read JPEG File.vi"("path to JPEG file"=w82) -> ("image data"=w81:T34)  [unwired: 8 in, 2 out]
  n4321 = call <vilib>:"Read JPEG File.vi"("path to JPEG file"=w39) -> ("image data"=w36:T34)  [unwired: 8 in, 2 out]
  n4322 = call <vilib>:"Read JPEG File.vi"("path to JPEG file"=w120) -> ("image data"=w119:T34)  [unwired: 8 in, 2 out]
  n4323 = call <vilib>:"Read JPEG File.vi"("path to JPEG file"=w68) -> ("image data"=w67:T34)  [unwired: 8 in, 2 out]
  n4324 = call <vilib>:"Read JPEG File.vi"("path to JPEG file"=w77) -> ("image data"=w78:T34)  [unwired: 8 in, 2 out]
  n4325 = call <vilib>:"Read JPEG File.vi"("path to JPEG file"=w83) -> ("image data"=w84:T34)  [unwired: 8 in, 2 out]
  n4326 = call <vilib>:"Read JPEG File.vi"("path to JPEG file"=w40) -> ("image data"=w41:T34)  [unwired: 8 in, 2 out]
  n4327 = call <vilib>:"Unflatten Pixmap.vi"("image data"=w305) -> ("24-bit pixmap"=w306:u32[][])  [unwired: 4 in, 6 out]
  n4328 = call <vilib>:"Read JPEG File.vi"("path to JPEG file"=w121) -> ("image data"=w122:T34)  [unwired: 8 in, 2 out]
  n4329 = call <vilib>:"Unflatten Pixmap.vi"("image data"=w128) -> ("24-bit pixmap"=w126:u32[][])  [unwired: 4 in, 6 out]
  n4330 = call <vilib>:"Read JPEG File.vi"("path to JPEG file"=w87) -> ("image data"=w90:T34)  [unwired: 8 in, 2 out]
  n4331 = call <vilib>:"Read JPEG File.vi"("path to JPEG file"=w86) -> ("image data"=w85:T34)  [unwired: 8 in, 2 out]
  n4332 = call <vilib>:"Unflatten Pixmap.vi"("image data"=w133) -> ("24-bit pixmap"=w125:u32[][])  [unwired: 4 in, 6 out]
  n4333 = call <vilib>:"Unflatten Pixmap.vi"("image data"=w113) -> ("24-bit pixmap"=w111:u32[][])  [unwired: 4 in, 6 out]
  n4334 = call <vilib>:"Unflatten Pixmap.vi"("image data"=w118) -> ("24-bit pixmap"=w110:u32[][])  [unwired: 4 in, 6 out]
  n4335 = call <vilib>:"Unflatten Pixmap.vi"("image data"=w248) -> ("24-bit pixmap"=w245:u32[][])  [unwired: 4 in, 6 out]
  n4336 = call <vilib>:"Unflatten Pixmap.vi"("image data"=w226) -> ("24-bit pixmap"=w225:u32[][])  [unwired: 4 in, 6 out]
  n4337 = call <vilib>:"Unflatten Pixmap.vi"("image data"=w251) -> ("24-bit pixmap"=w244:u32[][])  [unwired: 4 in, 6 out]
  n4338 = call <vilib>:"Unflatten Pixmap.vi"("image data"=w255) -> ("24-bit pixmap"=w232:u32[][])  [unwired: 4 in, 6 out]
  n4339 = call <vilib>:"Unflatten Pixmap.vi"("image data"=w260) -> ("24-bit pixmap"=w234:u32[][])  [unwired: 4 in, 6 out]
  n4340 = call <vilib>:"Unflatten Pixmap.vi"("image data"=w266) -> ("24-bit pixmap"=w243:u32[][])  [unwired: 4 in, 6 out]
  n4341 = call <vilib>:"Unflatten Pixmap.vi"("image data"=w252) -> ("24-bit pixmap"=w233:u32[][])  [unwired: 4 in, 6 out]
  n4342 = call <vilib>:"Unflatten Pixmap.vi"("image data"=w263) -> ("24-bit pixmap"=w235:u32[][])  [unwired: 4 in, 6 out]
  n4343 = call <vilib>:"Unflatten Pixmap.vi"("image data"=w269) -> ("24-bit pixmap"=w242:u32[][])  [unwired: 4 in, 6 out]
  n4344 = call <vilib>:"Unflatten Pixmap.vi"("image data"=w231) -> ("24-bit pixmap"=w224:u32[][])  [unwired: 4 in, 6 out]
  n4345 = call <vilib>:"Unflatten Pixmap.vi"("image data"=w486) -> ("24-bit pixmap"=w568:u32[][])  [unwired: 4 in, 6 out]
  n4346 = call <vilib>:"Unflatten Pixmap.vi"("image data"=w270) -> ("24-bit pixmap"=w240:u32[][])  [unwired: 4 in, 6 out]
  n4347 = call <vilib>:"Unflatten Pixmap.vi"("image data"=w221) -> ("24-bit pixmap"=w173:u32[][])  [unwired: 4 in, 6 out]
  n4348 = call <vilib>:"Unflatten Pixmap.vi"("image data"=w493) -> ("24-bit pixmap"=w567:u32[][])  [unwired: 4 in, 6 out]
  n4349 = call <vilib>:"Unflatten Pixmap.vi"("image data"=w218) -> ("24-bit pixmap"=w172:u32[][])  [unwired: 4 in, 6 out]
  n4350 = call <vilib>:"Unflatten Pixmap.vi"("image data"=w214) -> ("24-bit pixmap"=w171:u32[][])  [unwired: 4 in, 6 out]
  n4351 = call <vilib>:"Unflatten Pixmap.vi"("image data"=w209) -> ("24-bit pixmap"=w169:u32[][])  [unwired: 4 in, 6 out]
  n4352 = call <vilib>:"Unflatten Pixmap.vi"("image data"=w203) -> ("24-bit pixmap"=w167:u32[][])  [unwired: 4 in, 6 out]
  n4353 = call <vilib>:"Unflatten Pixmap.vi"("image data"=w289) -> ("24-bit pixmap"=w291:u32[][])  [unwired: 4 in, 6 out]
  n4354 = call <vilib>:"Unflatten Pixmap.vi"("image data"=w217) -> ("24-bit pixmap"=w170:u32[][])  [unwired: 4 in, 6 out]
  n4355 = call <vilib>:"Unflatten Pixmap.vi"("image data"=w206) -> ("24-bit pixmap"=w168:u32[][])  [unwired: 4 in, 6 out]
  n4356 = call <vilib>:"Unflatten Pixmap.vi"("image data"=w200) -> ("24-bit pixmap"=w166:u32[][])  [unwired: 4 in, 6 out]
  n4357 = call <vilib>:"Unflatten Pixmap.vi"("image data"=w428) -> ("24-bit pixmap"=w546:u32[][])  [unwired: 4 in, 6 out]
  n4358 = call <vilib>:"Unflatten Pixmap.vi"("image data"=w467) -> ("24-bit pixmap"=w559:u32[][])  [unwired: 4 in, 6 out]
  n4359 = call <vilib>:"Unflatten Pixmap.vi"("image data"=w295) -> ("24-bit pixmap"=w290:u32[][])  [unwired: 4 in, 6 out]
  n4360 = call <vilib>:"Unflatten Pixmap.vi"("image data"=w426) -> ("24-bit pixmap"=w547:u32[][])  [unwired: 4 in, 6 out]
  n4361 = call <vilib>:"Unflatten Pixmap.vi"("image data"=w199) -> ("24-bit pixmap"=w164:u32[][])  [unwired: 4 in, 6 out]
  n4362 = call <vilib>:"Unflatten Pixmap.vi"("image data"=w464) -> ("24-bit pixmap"=w558:u32[][])  [unwired: 4 in, 6 out]
  n4363 = call <vilib>:"Unflatten Pixmap.vi"("image data"=w281) -> ("24-bit pixmap"=w241:u32[][])  [unwired: 4 in, 6 out]
  n4364 = call <vilib>:"Unflatten Pixmap.vi"("image data"=w180) -> ("24-bit pixmap"=w175:u32[][])  [unwired: 4 in, 6 out]
  n4365 = call <vilib>:"Unflatten Pixmap.vi"("image data"=w414) -> ("24-bit pixmap"=w381:u32[][])  [unwired: 4 in, 6 out]
  n4366 = call <vilib>:"Unflatten Pixmap.vi"("image data"=w432) -> ("24-bit pixmap"=w545:u32[][])  [unwired: 4 in, 6 out]
  n4367 = call <vilib>:"Unflatten Pixmap.vi"("image data"=w417) -> ("24-bit pixmap"=w380:u32[][])  [unwired: 4 in, 6 out]
  n4368 = call <vilib>:"Unflatten Pixmap.vi"("image data"=w435) -> ("24-bit pixmap"=w544:u32[][])  [unwired: 4 in, 6 out]
  n4369 = call <vilib>:"Unflatten Pixmap.vi"("image data"=w176) -> ("24-bit pixmap"=w174:u32[][])  [unwired: 4 in, 6 out]
  n4370 = call <vilib>:"Unflatten Pixmap.vi"("image data"=w188) -> ("24-bit pixmap"=w165:u32[][])  [unwired: 4 in, 6 out]
  n4371 = call <vilib>:"Unflatten Pixmap.vi"("image data"=w93) -> ("24-bit pixmap"=w92:u32[][])  [unwired: 4 in, 6 out]
  n4372 = call <vilib>:"Unflatten Pixmap.vi"("image data"=w421) -> ("24-bit pixmap"=w383:u32[][])  [unwired: 4 in, 6 out]
  n4373 = call <vilib>:"Unflatten Pixmap.vi"("image data"=w98) -> ("24-bit pixmap"=w91:u32[][])  [unwired: 4 in, 6 out]
  n4374 = call <vilib>:"Unflatten Pixmap.vi"("image data"=w418) -> ("24-bit pixmap"=w382:u32[][])  [unwired: 4 in, 6 out]
  n4375 = call <vilib>:"Unflatten Pixmap.vi"("image data"=w63) -> ("24-bit pixmap"=w60:u32[][])  [unwired: 4 in, 6 out]
  n4376 = call <vilib>:"Unflatten Pixmap.vi"("image data"=w66) -> ("24-bit pixmap"=w59:u32[][])  [unwired: 4 in, 6 out]
  n4377 = call <vilib>:"Unflatten Pixmap.vi"("image data"=w70) -> ("24-bit pixmap"=w58:u32[][])  [unwired: 4 in, 6 out]
  n4378 = call <vilib>:"Unflatten Pixmap.vi"("image data"=w75) -> ("24-bit pixmap"=w56:u32[][])  [unwired: 4 in, 6 out]
  n4379 = call <vilib>:"Unflatten Pixmap.vi"("image data"=w81) -> ("24-bit pixmap"=w54:u32[][])  [unwired: 4 in, 6 out]
  n4380 = call <vilib>:"Unflatten Pixmap.vi"("image data"=w119) -> ("24-bit pixmap"=w109:u32[][])  [unwired: 4 in, 6 out]
  n4381 = call <vilib>:"Unflatten Pixmap.vi"("image data"=w67) -> ("24-bit pixmap"=w57:u32[][])  [unwired: 4 in, 6 out]
  n4382 = call <vilib>:"Unflatten Pixmap.vi"("image data"=w78) -> ("24-bit pixmap"=w55:u32[][])  [unwired: 4 in, 6 out]
  n4383 = call <vilib>:"Unflatten Pixmap.vi"("image data"=w84) -> ("24-bit pixmap"=w53:u32[][])  [unwired: 4 in, 6 out]
  n4384 = call <vilib>:"Unflatten Pixmap.vi"("image data"=w41) -> ("24-bit pixmap"=w33:u32[][])  [unwired: 4 in, 6 out]
  n4385 = call <vilib>:"Unflatten Pixmap.vi"("image data"=w122) -> ("24-bit pixmap"=w108:u32[][])  [unwired: 4 in, 6 out]
  n4386 = call <vilib>:"Unflatten Pixmap.vi"("image data"=w85) -> ("24-bit pixmap"=w51:u32[][])  [unwired: 4 in, 6 out]
  n4387 = call <vilib>:"Unflatten Pixmap.vi"("image data"=w36) -> ("24-bit pixmap"=w34:u32[][])  [unwired: 4 in, 6 out]
  n4388 = call <vilib>:"Unflatten Pixmap.vi"("image data"=w90) -> ("24-bit pixmap"=w52:u32[][])  [unwired: 4 in, 6 out]
  n4389 = while {
    tunnel: w585 -> [w5980]
    tunnel: w584 -> [w5981]
    tunnel: w583 -> [w5979]
    tunnel: w582 -> [w5978]
    tunnel: w581 -> [w5977]
    tunnel: w580 -> [w5976]
    tunnel: w579 -> [w5975]
    tunnel: w578 -> [w5974]
    tunnel: w577 -> [w5973]
    tunnel: w576 -> [w5972]
    tunnel: w575 -> [w5971]
    tunnel: w574 -> [w5970]
    tunnel: w573 -> [w5969]
    tunnel: w572 -> [w5968]
    tunnel: w362 -> [w5964]
    tunnel: w363 -> [w5965]
    tunnel: w345 -> [w5962]
    tunnel: w346 -> [w5963]
    tunnel: w344 -> [w5961]
    tunnel: w343 -> [w5960]
    tunnel: w329 -> [w5958]
    tunnel: w330 -> [w5959]
    tunnel: w321 -> [w5956]
    tunnel: w322 -> [w5957]
    tunnel: w315 -> [w5955]
    tunnel: w308 -> [w5954]
    tunnel: w307 -> [w5953]
    tunnel: w306 -> [w5952]
    tunnel: w296 -> [w5951]
    tunnel: w297 -> [w5950]
    stop <- FALSE stop-if-true
    n4390 = stacked-sequence {
      tunnel: w5980 -> [w6353 _ _]
      tunnel: [_ w6460 _] -> w5967
      tunnel: w5979 -> [w6386 _ _]
      tunnel: w5978 -> [w6384 _ _]
      tunnel: w5977 -> [w6379 _ _]
      tunnel: w5976 -> [w6333 _ _]
      tunnel: w5975 -> [w6374 _ _]
      tunnel: w5974 -> [w6365 _ _]
      tunnel: w5973 -> [w6356 _ _]
      tunnel: w5972 -> [w6355 _ _]
      tunnel: w5964 -> [w6342 _ _]
      tunnel: w5965 -> [w6341 _ _]
      frame #0 {
        n4391 = Build Array(FALSE ("element"), "chamber4 front piston open drum failed", "chamber4 front piston failed drum open", "chamber4 front piston open") -> (w6390:bool[])
        n4392 = Build Array(FALSE ("element"), "magnetron on ch4") -> (w6370:bool[])
        n4393 = Build Array(FALSE ("element"), "gv front open ch4_3", "gv front failed ch4_3") -> (w6382:bool[])
        n4394 = Build Array(FALSE ("element"), "magnetron water cooled on ch4", "magnetron water cooled failed_ch4") -> (w6357:bool[])
        n4395 = Build Array(FALSE ("element"), "Trns_gv_bp_on_ch4_front", "Trns_gv_bp_fail_ch4_front") -> (w6346:bool[])